vi "VP_RT_base.vi"() -> ()   [LabVIEW 2015] (continued)
                n36 = shared-variable ".\\Interloop communication.lvlib\\System command"(w61) -> ()  [unwired: 1 in, 1 out]
                n37 = local write "System Loop Type"(enum16{"Open Loop", "Closed Loop"}."Closed Loop" ("System Loop Type")) -> ()
              }
            }
            n38 = shared-variable "RT CompactRIO Target\\RT_EPICS_Shared_Variables.lvlib\\2iddVELO:VP:Base_Filename"() -> (w55:string)  [unwired: 1 in, 1 out]
            n39 = local read "EPICS Controller Type"() -> (w54:T2)
            n40 = local write "Fly Scan"(w48) -> ()
            n41 = local write "Controller Type"(w54) -> ()
            n42 = local write "Base name"(w55) -> ()
          }
        }
        "Snake Scan Reference FPGA or EPICS" <- w34
        "EPICS comms error" <- w29
        n43 = shared-variable ".\\Interloop communication.lvlib\\Base Filename"(w26) -> ()  [unwired: 1 in, 1 out]
        n44 = shared-variable ".\\Interloop communication.lvlib\\Command Loop Error"(w29) -> ()  [unwired: 1 in, 1 out]
        n45 = shared-variable ".\\Interloop communication.lvlib\\Fly Scan Flag"(w25) -> ()  [unwired: 1 in, 1 out]
      }
      frame True {
        n46 = shared-variable ".\\Interloop communication.lvlib\\System command"(Command_Enum."Stop System" ("System command")) -> (error out=w70:errorcluster)  [unwired: 1 in]
        n47 = shared-variable ".\\Interloop communication.lvlib\\New Command"(TRUE ("New Command"), error in=w70) -> ()  [unwired: 1 out]
      }
    }
    "Command Loop Iterations" <- w20
  }
  n48 = while {
    shift-right: [w87] -> _
    shift-left: TRUE -> [w88]
    i -> [w76]
    stop <- w80 stop-if-true
    # "Heartbeat Loop"
    n49 = shared-variable ".\\Interloop communication.lvlib\\EPICS command error"() -> (w74:errorcluster)  [unwired: 1 in, 1 out]
    n50 = shared-variable ".\\Interloop communication.lvlib\\Command Loop Error"() -> (w82:errorcluster)  [unwired: 1 in, 1 out]
    n51 = shared-variable ".\\Interloop communication.lvlib\\Readback Loop Error"() -> (w81:errorcluster)  [unwired: 1 in, 1 out]
    n52 = shared-variable ".\\Interloop communication.lvlib\\FPGA startup error"() -> (w79:errorcluster)  [unwired: 1 in, 1 out]
    n53 = shared-variable ".\\Interloop communication.lvlib\\Main Loop Error"() -> (w86:errorcluster)  [unwired: 1 in, 1 out]
    n54 = Not(x=w88) -> (.not. x?=w87:bool)
    "Heartbeat" <- w87
    n55 = call <vilib>:"RT LEDs.vi"("State"=3, "LED Num"=0) -> ("error out"=w75:errorcluster)  [unwired: 4 in, 1 out]
    n56 = Merge Errors(w75, w74, w82, w79, w86, w81) -> (w83:errorcluster)
    n57 = case shown="No Error" w83 {
      selector: w83 -> [w89 w91]
      tunnel: [u32 500 ("millisecond multiple") u32 100 ("millisecond multiple")] -> w85
      tunnel: [w89 w91] -> w84
      frame No Error {
      }
      frame Error {
      }
    }
    "RT error" <- w84
    n58 = local read "Stop System (Careful!!)"() -> (w80:bool)
    n59 = Wait Until Next ms Multiple(millisecond multiple=w85) -> ()  [unwired: 1 out]
    "Heartbeat Loop Iterations" <- w76
  }
  n60 = timed-loop {
    timing: w9 -> [_]
    timing-out: [_] -> w8
    shift-right: [w97] -> _
    shift-left: w4 -> [w94]
    shift-right: [w106] -> _
    shift-left: w2 -> [w98]
    shift-right: [w105] -> _
    shift-left: w1 -> [w99]
    shift-right: [w101] -> _
    shift-left: w3 -> [w102]
    i -> [w103]
    stop <- w108 stop-if-true
    # "Main Loop"
    n61 = node-c288() -> ()  [unwired: 1 in, 1 out]
    n62 = local read "Snake Scan Reference FPGA or EPICS"() -> (w96:enum16{"FPGA Snake Scan", "EPICS Snake Scan"})
    n63 = Format Into String(format string="%s", w94) -> (resulting string=w93:string)  [unwired: 2 in, 1 out]
    n64 = shared-variable "RT CompactRIO Target\\RT_EPICS_Shared_Variables.lvlib\\2iddVELO:VP:RT_State"(w93) -> ()  [unwired: 1 in, 1 out]
    n65 = case shown="\"Update Controller Info\"" w94 {
      tunnel: [w115 w136 w244 w331 w367 w482 w515 w528 w551 w592 w613 w683 w698 w710] -> w107
      tunnel: [FALSE ("Stop") FALSE ("Stop") FALSE ("Stop") FALSE ("Stop") FALSE ("Stop") FALSE ("Stop") FALSE ("Stop") FALSE ("Stop") _ FALSE ("Stop") FALSE ("Stop") FALSE ("Stop") FALSE ("Stop") TRUE ("Stop")] -> w108
      tunnel: [w118 w139 w243 w333 w365 w481 w514 w530 w542 w575 w639 w678 w693 w707] -> w106
      tunnel: [w110 w125 w242 w327 w364 w480 w513 w521 w541 w579 w637 w681 w692 w712] -> w105
      tunnel: w99 -> [w116 w134 w246 w328 w374 w484 w516 w531 w549 w577 w654 w673 w696 w716]
      tunnel: w98 -> [w117 w139 w245 w333 w375 w485 w517 w532 w550 w576 w640 w675 w702 w717]
      tunnel: w102 -> [w115 w136 w244 _ w367 w482 w515 w528 w551 w592 w614 w683 w698 _]
      tunnel: [i64 0 i64 0 i64 0 i64 50 i64 0 i64 0 i64 0 i64 0 i64 0 i64 250 w593 i64 0 i64 0 i64 0] -> w100
      tunnel: w96 -> [_ _ _ _ w361 w477 _ _ _ _ _ _ _ _]
      frame "Initialization", Default {
        n66 = xnode "Invoke Method"("FPGA VI Reference In"=w117, "error in"=w116, "Requested Depth"="Requested Depth") -> ("FPGA VI Reference Out"=w120:refnum<k20>, "error out"=w119:errorcluster, "Actual Depth"=→"Actual Depth":u32)
        n67 = xnode "Read/Write Control"("FPGA VI Reference In"=w120, "error in"=w119, "Datalog Time Period (uSec)"="Datalog Time Period (uSec)", "Datalog Cases"="Datalog Cases") -> ("FPGA VI Reference Out"=w112:refnum<k20>, "error out"=w111:errorcluster)
        n68 = xnode "Read/Write Control"("FPGA VI Reference In"=w112, "error in"=w111) -> ("FPGA VI Reference Out"=w118:refnum<k20>, "error out"=w110:errorcluster, "Wait error"=w109:errorcluster)
        "FPGA wait error" <- w109
        n69 = shared-variable ".\\Interloop communication.lvlib\\FPGA startup error"(w109) -> ()  [unwired: 1 in, 1 out]
      }
      frame "Import Controller coeffs" {
        n70 = case shown="\"PID\"" "Controller Type" {
          tunnel: ["file path soscoeff_zz1 Hinf" "file path soscoeff_zz1 PID"] -> w198
          tunnel: ["file path sos gain SF Controller_zz1 Hinf" "file path sos gain SF Controller_zz1 PID"] -> w196
          tunnel: ["file path soscoeff_yz1 Hinf" "file path soscoeff_zy1 PID"] -> w195
          tunnel: ["file path sos gain SF Controller_yz1 Hinf" "file path sos gain SF Controller_zy1 PID"] -> w194
          tunnel: ["file path soscoeff_yy1 Hinf" "file path soscoeff_yy1 PID"] -> w188
          tunnel: ["file path sos gain SF Controller_yy1 Hinf" "file path sos gain SF Controller_yy1 PID"] -> w187
          tunnel: ["file path soscoeff_zy1 Hinf" "file path soscoeff_yz1 PID"] -> w186
          tunnel: ["file path sos gain SF Controller_zy1 Hinf" "file path sos gain SF Controller_yz1 PID"] -> w185
          tunnel: ["file path soscoeff_xz1 Hinf" "file path soscoeff_zx1 PID"] -> w184
          tunnel: ["file path sos gain SF Controller_xz1 Hinf" "file path sos gain SF Controller_zx1 PID"] -> w183
          tunnel: ["file path soscoeff_xy1 Hinf" "file path soscoeff_yx1 PID"] -> w167
          tunnel: ["file path sos gain SF Controller_xy1 Hinf" "file path sos gain SF Controller_yx1 PID"] -> w166
          tunnel: ["file path sos gain SF Controller_zx1 Hinf" "file path sos gain SF Controller_xz1 PID"] -> w160
          tunnel: ["file path soscoeff_zx1 Hinf" "file path soscoeff_xz1 PID"] -> w159
          tunnel: ["file path sos gain SF Controller_xx1 Hinf" "file path sos gain SF Controller_xx1 PID"] -> w153
          tunnel: ["file path soscoeff_xx1 Hinf" "file path soscoeff_xx1 PID"] -> w152
          tunnel: ["file path soscoeff_yx1 Hinf" "file path soscoeff_xy1 PID"] -> w151
          tunnel: ["file path sos gain SF Controller_yx1 Hinf" "file path sos gain SF Controller_xy1 PID"] -> w150
          frame "H-infinity", Default {
          }
          frame "PID" {
          }
        }
        n71 = call "Read_coeff.vi"("error in (no error)"=w134, "sos gain SF controller file path"=w153, "sos coeff file path"=w152) -> ("b02(2)"=→"b02(2) xx1c":fxp<+/-,64,9>[], "b01(2)"=→"b01(2) xx1c":fxp<+/-,64,9>[], "-a02(2)"=→"-a02(2) xx1c":fxp<+/-,64,9>[], "-a01(2)"=→"-a01(2) xx1c":fxp<+/-,64,9>[], "error out"=w133:errorcluster, "sos gain SF Controller"=→"sos gain SF Controller xx1c":fxp<+/-,42,9>)  [unwired: 3 in]
        n72 = call "Read_coeff.vi"("error in (no error)"=w133, "sos gain SF controller file path"=w166, "sos coeff file path"=w167) -> ("b02(2)"=→"b02(2) xy1c":fxp<+/-,64,9>[], "b01(2)"=→"b01(2) xy1c":fxp<+/-,64,9>[], "-a02(2)"=→"-a02(2) xy1c":fxp<+/-,64,9>[], "-a01(2)"=→"-a01(2) xy1c":fxp<+/-,64,9>[], "error out"=w132:errorcluster, "sos gain SF Controller"=→"sos gain SF Controller xy1c":fxp<+/-,42,9>)  [unwired: 3 in]
        n73 = call "Read_coeff.vi"("error in (no error)"=w132, "sos gain SF controller file path"=w183, "sos coeff file path"=w184) -> ("b02(2)"=→"b02(2) xz1c":fxp<+/-,64,9>[], "b01(2)"=→"b01(2) xz1c":fxp<+/-,64,9>[], "-a02(2)"=→"-a02(2) xz1c":fxp<+/-,64,9>[], "-a01(2)"=→"-a01(2) xz1c":fxp<+/-,64,9>[], "error out"=w131:errorcluster, "sos gain SF Controller"=→"sos gain SF Controller xz1c":fxp<+/-,42,9>)  [unwired: 3 in]
        n74 = call "Read_coeff.vi"("error in (no error)"=w131, "sos gain SF controller file path"=w150, "sos coeff file path"=w151) -> ("b02(2)"=→"b02(2) yx1c":fxp<+/-,64,9>[], "b01(2)"=→"b01(2) yx1c":fxp<+/-,64,9>[], "-a02(2)"=→"-a02(2) yx1c":fxp<+/-,64,9>[], "-a01(2)"=→"-a01(2) yx1c":fxp<+/-,64,9>[], "error out"=w130:errorcluster, "sos gain SF Controller"=→"sos gain SF Controller yx1c":fxp<+/-,42,9>)  [unwired: 3 in]
        n75 = call "Read_coeff.vi"("error in (no error)"=w130, "sos gain SF controller file path"=w187, "sos coeff file path"=w188) -> ("b02(2)"=→"b02(2) yy1c":fxp<+/-,64,9>[], "b01(2)"=→"b01(2) yy1c":fxp<+/-,64,9>[], "-a02(2)"=→"-a02(2) yy1c":fxp<+/-,64,9>[], "-a01(2)"=→"-a01(2) yy1c":fxp<+/-,64,9>[], "error out"=w129:errorcluster, "sos gain SF Controller"=→"sos gain SF Controller yy1c":fxp<+/-,42,9>)  [unwired: 3 in]
        n76 = call "Read_coeff.vi"("error in (no error)"=w129, "sos gain SF controller file path"=w194, "sos coeff file path"=w195) -> ("b02(2)"=→"b02(2) yz1c":fxp<+/-,64,9>[], "b01(2)"=→"b01(2) yz1c":fxp<+/-,64,9>[], "-a02(2)"=→"-a02(2) yz1c":fxp<+/-,64,9>[], "-a01(2)"=→"-a01(2) yz1c":fxp<+/-,64,9>[], "error out"=w128:errorcluster, "sos gain SF Controller"=→"sos gain SF Controller yz1c":fxp<+/-,42,9>)  [unwired: 3 in]
        n77 = call "Read_coeff.vi"("error in (no error)"=w128, "sos gain SF controller file path"=w160, "sos coeff file path"=w159) -> ("b02(2)"=→"b02(2) zx1c":fxp<+/-,64,9>[], "b01(2)"=→"b01(2) zx1c":fxp<+/-,64,9>[], "-a02(2)"=→"-a02(2) zx1c":fxp<+/-,64,9>[], "-a01(2)"=→"-a01(2) zx1c":fxp<+/-,64,9>[], "error out"=w127:errorcluster, "sos gain SF Controller"=→"sos gain SF Controller zx1c":fxp<+/-,42,9>)  [unwired: 3 in]
        n78 = call "Read_coeff.vi"("error in (no error)"=w127, "sos gain SF controller file path"=w185, "sos coeff file path"=w186) -> ("b02(2)"=→"b02(2) zy1c":fxp<+/-,64,9>[], "b01(2)"=→"b01(2) zy1c":fxp<+/-,64,9>[], "-a02(2)"=→"-a02(2) zy1c":fxp<+/-,64,9>[], "-a01(2)"=→"-a01(2) zy1c":fxp<+/-,64,9>[], "error out"=w126:errorcluster, "sos gain SF Controller"=→"sos gain SF Controller zy1c":fxp<+/-,42,9>)  [unwired: 3 in]
        n79 = call "Read_coeff.vi"("error in (no error)"=w126, "sos gain SF controller file path"=w196, "sos coeff file path"=w198) -> ("b02(2)"=→"b02(2) zz1c":fxp<+/-,64,9>[], "b01(2)"=→"b01(2) zz1c":fxp<+/-,64,9>[], "-a02(2)"=→"-a02(2) zz1c":fxp<+/-,64,9>[], "-a01(2)"=→"-a01(2) zz1c":fxp<+/-,64,9>[], "error out"=w125:errorcluster, "sos gain SF Controller"=→"sos gain SF Controller zz1c":fxp<+/-,42,9>)  [unwired: 3 in]
        "Coeff file import error" <- w125
      }
      frame "Update Controller Info" {
        n80 = local read "sos gain SF Controller yy1c"() -> (w305:fxp<+/-,42,9>)
        n81 = local read "sos gain SF Controller yz1c"() -> (w254:fxp<+/-,42,9>)
        n82 = local read "sos gain SF Controller yx1c"() -> (w293:fxp<+/-,42,9>)
        n83 = local read "sos gain SF Controller xy1c"() -> (w279:fxp<+/-,42,9>)
        n84 = local read "sos gain SF Controller zy1c"() -> (w284:fxp<+/-,42,9>)
        n85 = local read "sos gain SF Controller xz1c"() -> (w268:fxp<+/-,42,9>)
        n86 = local read "sos gain SF Controller xx1c"() -> (w310:fxp<+/-,42,9>)
        n87 = local read "sos gain SF Controller zz1c"() -> (w303:fxp<+/-,42,9>)
        n88 = local read "sos gain SF Controller zx1c"() -> (w289:fxp<+/-,42,9>)
        n89 = local read "-a01(2) yy1c"() -> (w309:fxp<+/-,64,9>[])
        n90 = local read "-a02(2) yy1c"() -> (w308:fxp<+/-,64,9>[])
        n91 = local read "-a01(2) yz1c"() -> (w273:fxp<+/-,64,9>[])
        n92 = local read "-a02(2) yz1c"() -> (w274:fxp<+/-,64,9>[])
        n93 = local read "-a01(2) yx1c"() -> (w294:fxp<+/-,64,9>[])
        n94 = local read "-a02(2) yx1c"() -> (w290:fxp<+/-,64,9>[])
        n95 = local read "-a01(2) xy1c"() -> (w275:fxp<+/-,64,9>[])
        n96 = local read "-a02(2) xy1c"() -> (w276:fxp<+/-,64,9>[])
        n97 = local read "-a01(2) zy1c"() -> (w280:fxp<+/-,64,9>[])
        n98 = local read "-a02(2) zy1c"() -> (w281:fxp<+/-,64,9>[])
        n99 = local read "-a01(2) xz1c"() -> (w272:fxp<+/-,64,9>[])
        n100 = local read "-a02(2) xz1c"() -> (w271:fxp<+/-,64,9>[])
        n101 = local read "-a01(2) xx1c"() -> (w314:fxp<+/-,64,9>[])
        n102 = local read "-a02(2) xx1c"() -> (w313:fxp<+/-,64,9>[])
        n103 = local read "-a01(2) zz1c"() -> (w304:fxp<+/-,64,9>[])
        n104 = local read "-a02(2) zz1c"() -> (w300:fxp<+/-,64,9>[])
        n105 = local read "-a01(2) zx1c"() -> (w285:fxp<+/-,64,9>[])
        n106 = local read "-a02(2) zx1c"() -> (w286:fxp<+/-,64,9>[])
        n107 = local read "b01(2) yy1c"() -> (w307:fxp<+/-,64,9>[])
        n108 = local read "b02(2) yy1c"() -> (w306:fxp<+/-,64,9>[])
        n109 = local read "b01(2) yz1c"() -> (w248:fxp<+/-,64,9>[])
        n110 = local read "b02(2) yz1c"() -> (w247:fxp<+/-,64,9>[])
        n111 = local read "b01(2) yx1c"() -> (w291:fxp<+/-,64,9>[])
        n112 = local read "b02(2) yx1c"() -> (w292:fxp<+/-,64,9>[])
        n113 = local read "b01(2) xy1c"() -> (w277:fxp<+/-,64,9>[])
        n114 = local read "b02(2) xy1c"() -> (w278:fxp<+/-,64,9>[])
        n115 = local read "b01(2) zy1c"() -> (w282:fxp<+/-,64,9>[])
        n116 = local read "b02(2) zy1c"() -> (w283:fxp<+/-,64,9>[])
        n117 = local read "b01(2) xz1c"() -> (w270:fxp<+/-,64,9>[])
        n118 = local read "b02(2) xz1c"() -> (w269:fxp<+/-,64,9>[])
        n119 = local read "b01(2) xx1c"() -> (w312:fxp<+/-,64,9>[])
        n120 = local read "b02(2) xx1c"() -> (w311:fxp<+/-,64,9>[])
        n121 = local read "b01(2) zz1c"() -> (w301:fxp<+/-,64,9>[])
        n122 = local read "b02(2) zz1c"() -> (w302:fxp<+/-,64,9>[])
        n123 = local read "b01(2) zx1c"() -> (w287:fxp<+/-,64,9>[])
        n124 = local read "b02(2) zx1c"() -> (w288:fxp<+/-,64,9>[])
        n125 = Or(x="Optics Z Reset", y="Reset All") -> (x .or. y?=w267:bool)
        n126 = Or(x="Sample Z Reset", y="Reset All") -> (x .or. y?=w264:bool)
        n127 = Or(x="Optics X Reset", y="Reset All") -> (x .or. y?=w298:bool)
        n128 = Or(x="Optics Y Reset", y="Reset All") -> (x .or. y?=w296:bool)
        n129 = Or(x="Sample X Reset", y="Reset All") -> (x .or. y?=w266:bool)
        n130 = Or(x="Sample Y Reset", y="Reset All") -> (x .or. y?=w265:bool)
        n131 = xnode "Read/Write Control"("FPGA VI Reference In"=w245, "error in"=w246, "Wait timer (ms)"="FPGA Wait Timer (ms)", "Controller Time Period (uSec)"="Controller Time Period (uSec)", "Controller Output Time Period (uSec)"="Controller Output Time Period (uSec)", "System Loop Type"="System Loop Type", "Controller Output Upper Limit"="Controller Output Upper Limit", "Controller Output Lower Limit"="Controller Output Lower Limit", "X-Stage nm to V Scaling"="X-Stage nm to V Scaling", "X-Stage Scaling Direction"="X-Stage Scaling Direction", "Y-Stage nm to V Scaling"="Y-Stage nm to V Scaling", "Z-Stage nm to V Scaling"="Z-Stage nm to V Scaling", "Plant Output Time Period (uSec)"="Plant Output Time Period (uSec)", "Reset Optics X"=w298, "Reset Optics Y"=w296, "Reset Optics Z"=w267, "Reset Sample X"=w266, "Reset Sample Y"=w265, "Reset Sample Z"=w264, "Optics X Stage Resolution (nm)"="Optics X Stage Resolution (nm)", "Optics Y Stage Resolution (nm)"="Optics Y Stage Resolution (nm)", "Optics Z Stage Resolution (nm)"="Optics Z Stage Resolution (nm)", "Sample X Stage Resolution (nm)"="Sample X Stage Resolution (nm)", "Sample Y Stage Resolution (nm)"="Sample Y Stage Resolution (nm)", "Sample Z Stage Resolution (nm)"="Sample Z Stage Resolution (nm)", "Scaling mV to V"="Scaling mV to V", "-a01(2) xx1"=w314, "-a02(2) xx1"=w313, "b01(2) xx1"=w312, "b02(2) xx1"=w311, "sos gain SF Controller xx1"=w310, "-a01(2) yy1"=w309, "-a02(2) yy1"=w308, "b01(2) yy1"=w307, "b02(2) yy1"=w306, "sos gain SF Controller yy1"=w305, "-a01(2) zz1"=w304, "-a02(2) zz1"=w300, "b01(2) zz1"=w301, "b02(2) zz1"=w302, "sos gain SF Controller zz1"=w303, "-a01(2) yx1"=w294, "-a02(2) yx1"=w290, "b01(2) yx1"=w291, "b02(2) yx1"=w292, "sos gain SF Controller yx1"=w293, "-a01(2) zx1"=w285, "-a02(2) zx1"=w286, "b01(2) zx1"=w287, "b02(2) zx1"=w288, "sos gain SF Controller zx1"=w289, "-a01(2) xy1"=w275, "-a02(2) xy1"=w276, "b01(2) xy1"=w277, "b02(2) xy1"=w278, "sos gain SF Controller xy1"=w279, "-a01(2) zy1"=w280, "-a02(2) zy1"=w281, "b01(2) zy1"=w282, "b02(2) zy1"=w283, "sos gain SF Controller zy1"=w284, "-a01(2) xz1"=w272, "-a02(2) xz1"=w271, "b01(2) xz1"=w270, "b02(2) xz1"=w269, "sos gain SF Controller xz1"=w268, "-a01(2) yz1"=w273, "-a02(2) yz1"=w274, "b01(2) yz1"=w248, "b02(2) yz1"=w247, "sos gain SF Controller yz1"=w254, "Analog Input Time Period (uSec)"="Analog Input Time Period (uSec)", "Optics and or Sample Stage"="Optics and or Sample Stage", "Y-Stage Scaling Direction"="Y-Stage Scaling Direction", "Z-Stage Scaling Direction"="Z-Stage Scaling Direction") -> ("FPGA VI Reference Out"=w243:refnum<k20>, "error out"=w242:errorcluster)
      }
      frame "Wait" {
        n132 = shared-variable ".\\Interloop communication.lvlib\\New Command"() -> (w332:bool, error out=w330:errorcluster)  [unwired: 1 in]
        n133 = case shown="True" w332 {
          tunnel: [w335 w336] -> w331
          tunnel: w330 -> [_ w340]
          tunnel: w328 -> [w334 w338]
          tunnel: [w334 w337] -> w327
          frame False {
            w335 = T11[] [enum."Wait"] items=["Initialization", "Import Controller coeffs", "Update Controller Info", "Wait", "Update Reference Info", "Update Detector Trigger Info", "Update Datalog Info", "Check FPGA Status", "Pre-Scan", "Start Scan", "Step Scanning", "Fly Scanning", "End Scan", "Restart FPGA", "Stop FPGA"]
          }
          frame True {
            n134 = shared-variable ".\\Interloop communication.lvlib\\System command"() -> (w339:T8)  [unwired: 1 in, 1 out]
            "Last Command Executed" <- w339
            n135 = case shown="\"Scan\"" w339 {
              tunnel: [w344 w347 w350 w353 w356 w360] -> w336
              tunnel: w338 -> [w343 w346 w349 w352 w355 w359]
              tunnel: [w342 w345 w348 w351 w354 w358] -> w337
              frame "Re-Initialize ", Default {
                w344 = T11[] [enum."Initialization", enum."Import Controller coeffs", enum."Update Controller Info", enum."Wait"] items=["Initialization", "Import Controller coeffs", "Update Controller Info", "Wait", "Update Reference Info", "Update Detector Trigger Info", "Update Datalog Info", "Check FPGA Status", "Pre-Scan", "Start Scan", "Step Scanning", "Fly Scanning", "End Scan", "Restart FPGA", "Stop FPGA"]
                n136 = call <vilib>:"Clear Errors.vi"("error in (no error)"=w343) -> ("error out"=w342:errorcluster)  [unwired: 5 in, 1 out]
              }
              frame "Update Scan Settings" {
                w347 = T11[] [enum."Update Reference Info", enum."Update Detector Trigger Info", enum."Update Datalog Info", enum."Wait"] items=["Initialization", "Import Controller coeffs", "Update Controller Info", "Wait", "Update Reference Info", "Update Detector Trigger Info", "Update Datalog Info", "Check FPGA Status", "Pre-Scan", "Start Scan", "Step Scanning", "Fly Scanning", "End Scan", "Restart FPGA", "Stop FPGA"]
                n137 = call <vilib>:"Clear Errors.vi"("error in (no error)"=w346) -> ("error out"=w345:errorcluster)  [unwired: 5 in, 1 out]
              }
              frame "Scan" {
                w350 = T11[] [enum."Update Reference Info", enum."Update Detector Trigger Info", enum."Update Datalog Info", enum."Pre-Scan", enum."Start Scan", enum."Fly Scanning", enum."End Scan", enum."Wait"] items=["Initialization", "Import Controller coeffs", "Update Controller Info", "Wait", "Update Reference Info", "Update Detector Trigger Info", "Update Datalog Info", "Check FPGA Status", "Pre-Scan", "Start Scan", "Step Scanning", "Fly Scanning", "End Scan", "Restart FPGA", "Stop FPGA"]
                n138 = call <vilib>:"Clear Errors.vi"("error in (no error)"=w349) -> ("error out"=w348:errorcluster)  [unwired: 5 in, 1 out]
              }
              frame "Stop Scan" {
                w353 = T11[] [enum."End Scan", enum."Wait"] items=["Initialization", "Import Controller coeffs", "Update Controller Info", "Wait", "Update Reference Info", "Update Detector Trigger Info", "Update Datalog Info", "Check FPGA Status", "Pre-Scan", "Start Scan", "Step Scanning", "Fly Scanning", "End Scan", "Restart FPGA", "Stop FPGA"]
                n139 = call <vilib>:"Clear Errors.vi"("error in (no error)"=w352) -> ("error out"=w351:errorcluster)  [unwired: 5 in, 1 out]
              }
              frame "Restart FPGA" {
                w356 = T11[] [enum."Restart FPGA", enum."Initialization", enum."Import Controller coeffs", enum."Update Controller Info", enum."Wait"] items=["Initialization", "Import Controller coeffs", "Update Controller Info", "Wait", "Update Reference Info", "Update Detector Trigger Info", "Update Datalog Info", "Check FPGA Status", "Pre-Scan", "Start Scan", "Step Scanning", "Fly Scanning", "End Scan", "Restart FPGA", "Stop FPGA"]
                n140 = call <vilib>:"Clear Errors.vi"("error in (no error)"=w355) -> ("error out"=w354:errorcluster)  [unwired: 5 in, 1 out]
              }
              frame "Stop System" {
                w360 = T11[] [enum."Stop FPGA"] items=["Initialization", "Import Controller coeffs", "Update Controller Info", "Wait", "Update Reference Info", "Update Detector Trigger Info", "Update Datalog Info", "Check FPGA Status", "Pre-Scan", "Start Scan", "Step Scanning", "Fly Scanning", "End Scan", "Restart FPGA", "Stop FPGA"]
                n141 = call <vilib>:"Clear Errors.vi"("error in (no error)"=w359) -> ("error out"=w358:errorcluster)  [unwired: 5 in, 1 out]
                n142 = local write "Stop System (Careful!!)"(TRUE ("Stop")) -> ()
              }
            }
            n143 = shared-variable ".\\Interloop communication.lvlib\\New Command"(FALSE ("New Command"), error in=w340) -> ()  [unwired: 1 out]
          }
        }
      }
      frame "Update Reference Info" {
        w427 = errorcluster {"status"=FALSE, "code"=0, "source"=""}  # error in (no error)
        w430 = errorcluster {"status"=FALSE, "code"=0, "source"=""}  # error in (no error)
        w444 = errorcluster {"status"=FALSE, "code"=0, "source"=""}  # error in (no error)
        w423 = 40000000.0  # FPGA clock rate (Hz)
        n144 = local read "Measured Z Reference Time Period (Ticks)"() -> (w366:u32)
        n145 = case shown="\"EPICS Snake Scan\"" w361 {
          tunnel: ["X Ramp Start (nm)" w460] -> w382
          tunnel: ["X Ramp End (nm)" w459] -> w381
          tunnel: ["Y Ramp Start (nm)" w458] -> w380
          tunnel: ["Y Ramp End (nm)" w457] -> w379
          tunnel: ["Y Step Size (nm)" w461] -> w378
          tunnel: ["X Step Size (nm)" w464] -> w377
          tunnel: [w452 w462] -> w376
          tunnel: ["Y Step Size (nm)" w461] -> w373
          tunnel: ["X Ramp Start (nm)" w460] -> w372
          tunnel: ["X Ramp End (nm)" w459] -> w371
          tunnel: ["Y Ramp Start (nm)" w458] -> w370
          tunnel: ["Y Ramp End (nm)" w457] -> w369
          frame "FPGA Snake Scan", Default {
            n146 = local read "DT Frequency (Hz)"() -> (w452:dbl)
          }
          frame "EPICS Snake Scan" {
            w463 = fxp<+/-,16,16> 0.0 ("fixed-point type")
            n147 = shared-variable "RT CompactRIO Target\\RT_EPICS_Shared_Variables.lvlib\\2iddVELO:VP:Trigger_Freq_Hz"() -> (w462:dbl)  [unwired: 1 in, 1 out]
            "2iddVELO:VP:Trigger_Freq_Hz" <- w462
            n148 = shared-variable "RT CompactRIO Target\\RT_EPICS_Shared_Variables.lvlib\\2iddVELO:VP:Y_Step_Size_nm"() -> (w466:dbl)  [unwired: 1 in, 1 out]
            "2iddVELO:VP:Y_Step_Size_nm" <- w466
            n149 = shared-variable "RT CompactRIO Target\\RT_EPICS_Shared_Variables.lvlib\\2iddVELO:VP:X_Step_Size_nm"() -> (w465:dbl)  [unwired: 1 in, 1 out]
            "2iddVELO:VP:X_Step_Size_nm" <- w465
            n150 = shared-variable "RT CompactRIO Target\\RT_EPICS_Shared_Variables.lvlib\\2iddVELO:VP:Y_Start_nm"() -> (w467:dbl)  [unwired: 1 in, 1 out]
            n151 = shared-variable "RT CompactRIO Target\\RT_EPICS_Shared_Variables.lvlib\\2iddVELO:VP:Y_End_nm"() -> (w456:dbl)  [unwired: 1 in, 1 out]
            n152 = shared-variable "RT CompactRIO Target\\RT_EPICS_Shared_Variables.lvlib\\2iddVELO:VP:X_Start_nm"() -> (w469:dbl)  [unwired: 1 in, 1 out]
            "2iddVELO:VP:X_Start_nm" <- w469
            n153 = shared-variable "RT CompactRIO Target\\RT_EPICS_Shared_Variables.lvlib\\2iddVELO:VP:X_End_nm"() -> (w468:dbl)  [unwired: 1 in, 1 out]
            "2iddVELO:VP:X_End_nm" <- w468
            n154 = Negate(x=w456) -> (-x=w455:dbl)
            "2iddVELO:VP:Y_End_nm" <- w455
            n155 = Negate(x=w467) -> (-x=w454:dbl)
            "2iddVELO:VP:Y_Start_nm" <- w454
            n156 = To Fixed-Point(fixed-point type=w463, number=w469) -> (fixed-point=w460:fxp<+/-,16,16>)
            n157 = To Fixed-Point(fixed-point type=w463, number=w468) -> (fixed-point=w459:fxp<+/-,16,16>)
            n158 = To Fixed-Point(fixed-point type=w463, number=w454) -> (fixed-point=w458:fxp<+/-,16,16>)
            n159 = To Fixed-Point(fixed-point type=w463, number=w455) -> (fixed-point=w457:fxp<+/-,16,16>)
            n160 = To Fixed-Point(fixed-point type=w463, number=w466) -> (fixed-point=w461:fxp<+/-,16,16>)
            n161 = To Fixed-Point(fixed-point type=w463, number=w465) -> (fixed-point=w464:fxp<+/-,16,16>)
          }
        }
        n162 = local read "Y Ramp Period (usec)"() -> (w384:fxp<+,24,24>)
        n163 = shared-variable ".\\Interloop communication.lvlib\\Fly Scan Flag"() -> (w368:bool)  [unwired: 1 in, 1 out]
        n164 = case shown="\"Sawtooth Wave\"" "Z Reference Wave Selection" {
          tunnel: "Z frequency (Hz)" -> [w470 w471 w473 w475 w476]
          tunnel: [w470 w471 w472 w475 w476] -> w405
          tunnel: w366 -> [_ _ w474 _ _]
          frame "Constant", Default {
          }
          frame "Sine Wave" {
          }
          frame "Sawtooth Wave" {
            n165 = Multiply(x=w474, y=w473) -> (x*y=w472:dbl)
          }
          frame "Square Wave" {
          }
          frame "Filtered White Noise" {
          }
        }
        n166 = call <vilib>:"Normalize Signal Generation Parameters.vi"("frequency (Hz)"="X frequency (Hz)", "FPGA clock rate (Hz)"=w423, "phase offset (deg)"="X phase offset (deg)", "error in (no error)"=w444) -> ("frequency (periods/tick)"=w443:fxp<+,32,0>, "phase offset (periods)"=w433:fxp<+,32,0>, "error out"=→"error out (Sig Gen)":errorcluster)  [unwired: 6 in, 3 out]
        "X frequency (periods/tick)" <- w443
        "X phase offset (periods)" <- w433
        n167 = call <vilib>:"Normalize Signal Generation Parameters.vi"("frequency (Hz)"="Y frequency (Hz)", "FPGA clock rate (Hz)"=w423, "phase offset (deg)"="Y phase offset (deg)", "error in (no error)"=w430) -> ("frequency (periods/tick)"=w426:fxp<+,32,0>, "phase offset (periods)"=w425:fxp<+,32,0>, "error out"=→"error out (Sig Gen) 2":errorcluster)  [unwired: 6 in, 3 out]
        "Y frequency (periods/tick)" <- w426
        "Y phase offset (periods)" <- w425
        n168 = call <vilib>:"Normalize Signal Generation Parameters.vi"("frequency (Hz)"=w405, "FPGA clock rate (Hz)"=w423, "phase offset (deg)"="Z phase offset (deg)", "error in (no error)"=w427) -> ("frequency (periods/tick)"=w424:fxp<+,32,0>, "phase offset (periods)"=w416:fxp<+,32,0>, "error out"=→"error out (Sig Gen) 3":errorcluster)  [unwired: 6 in, 3 out]
        "Z frequency (periods/tick)" <- w424
        "Z phase offset (periods)" <- w416
        n169 = local read "X Ramp Period (usec)"() -> (w383:fxp<+,24,24>)
        n170 = xnode "Read/Write Control"("FPGA VI Reference In"=w375, "error in"=w374, "X Reference Time Period (uSec)"="X Reference Time Period (uSec)", "Y Reference Time Period (uSec)"="Y Reference Time Period (uSec)", "Z Reference Time Period (uSec)"="Z Reference Time Period (uSec)", "X Reference Wave Selection"="X Reference Wave Selection", "Y Reference Wave Selection"="Y Reference Wave Selection", "Z Reference Wave Selection"="Z Reference Wave Selection", "X Reference Reset"="X Reference Reset", "Y Reference Reset"="Y Reference Reset", "Z Reference Reset"="Z Reference Reset", "X Reference Amplitude (nm)"="X Reference Amplitude (nm)", "Y Reference Amplitude (nm)"="Y Reference Amplitude (nm)", "Z Reference Amplitude (nm)"="Z Reference Amplitude (nm)", "X Frequency (periods/tick)"=w443, "X Phase Offset (periods)"=w433, "Y Frequency (periods/tick)"=w426, "Y Phase Offset (periods)"=w425, "Z Frequency (periods/tick)"=w424, "Z Phase Offset (periods)"=w416, "X Reference DC Offset (nm)"="X Reference DC Offset (nm)", "Y Reference DC Offset (nm)"="Y Reference DC Offset (nm)", "Z Reference DC Offset (nm)"="Z Reference DC Offset (nm)", "X White Noise Amplitude"="X White Noise Amplitude", "X White Noise Seed"="X White Noise Seed", "Y White Noise Amplitude"="Y White Noise Amplitude", "Y White Noise Seed"="Y White Noise Seed", "Z White Noise Amplitude"="Z White Noise Amplitude", "Z White Noise Seed"="Z White Noise Seed", "Mod 3 AI0 V to nm Scaling"="Mod 3 AI0 V to nm Scaling", "Mod 3 AI1 V to nm Scaling"="Mod 3 AI1 V to nm Scaling", "Mod 3 AI2 V to nm Scaling"="Mod 3 AI2 V to nm Scaling", "X Ramp Period (usec)"=w383, "X Ramp Start (nm)"=w382, "X Ramp End (nm)"=w381, "X Start Marker (nm)"="X Start Marker (nm)", "Fly Scan"=w368, "Y Ramp Period (usec)"=w384, "Y Ramp Start (nm)"=w380, "Y Ramp End (nm)"=w379, "Y Ramp Drop Size (nm)"=w378, "Y Start Marker (nm)"="Y Start Marker (nm)") -> ("FPGA VI Reference Out"=w365:refnum<k20>, "error out"=w364:errorcluster)
        n171 = Subtract(x=w370, y=w369) -> (x-y=w400:fxp<+/-,17,17>)
        n172 = Subtract(x=w372, y=w371) -> (x-y=w398:fxp<+/-,17,17>)
        n173 = Absolute Value(x=w400) -> (abs(x)=w391:fxp<+,16,16>)
        n174 = Absolute Value(x=w398) -> (abs(x)=w397:fxp<+,16,16>)
        n175 = Divide(x=w397, y=w377) -> (x/y=w395:fxp<+/-,33,17>)
        "# of Points per Line" <- w395
        n176 = Divide(x=w395, y=w376) -> (x/y=w387:dbl)
        "sec per line" <- w387
        n177 = Divide(x=w391, y=w373) -> (x/y=w392:fxp<+/-,33,17>)
        n178 = Add(x=w392, y=fxp<+,16,16> 1.0) -> (x+y=w386:fxp<+/-,34,18>)
        "# of Hor Lines" <- w386
        n179 = Multiply(x=w387, y=1000000.0) -> (x*y=w390:dbl)
        "X Ramp Period DBL (usec)" <- w390
        n180 = Reciprocal(x=w387) -> (1/x=→"line per sec (Hz)":dbl)
        n181 = To Fixed-Point(fixed-point type=fxp<+,24,24> 0.0, number=w390) -> (fixed-point=→"X Ramp Period (usec)" →"Y Ramp Period (usec)":fxp<+,24,24>)
        n182 = Multiply(x=w387, y=w386) -> (x*y=→"Total Scan Time (sec)":dbl)
        n183 = Multiply(x=w386, y=w395) -> (x*y=→"# Total Trigger Points":fxp<+/-,64,34>)
      }
      frame "Update Detector Trigger Info" {
        w491 = 40000000.0  # FPGA clock rate (Hz)
        w493 = errorcluster {"status"=FALSE, "code"=0, "source"=""}  # error in (no error)
        n184 = case shown="\"EPICS Snake Scan\"" w477 {
          tunnel: ["DT Frequency (Hz)" w510] -> w492
          tunnel: ["DT duty cycle (%)" w509] -> w486
          frame "FPGA Snake Scan", Default {
          }
          frame "EPICS Snake Scan" {
            n185 = shared-variable "RT CompactRIO Target\\RT_EPICS_Shared_Variables.lvlib\\2iddVELO:VP:Trig_DutyCycle_Per"() -> (w509:dbl)  [unwired: 1 in, 1 out]
            "2iddVELO:VP:Trig_DutyCycle_Per" <- w509
            n186 = shared-variable "RT CompactRIO Target\\RT_EPICS_Shared_Variables.lvlib\\2iddVELO:VP:Trigger_Freq_Hz"() -> (w510:dbl)  [unwired: 1 in, 1 out]
          }
        }
        "Trigger Frequency (Hz)" <- w492
        "Trigger Duty Cycle (%)" <- w486
        n187 = call <vilib>:"Normalize Signal Generation Parameters.vi"("frequency (Hz)"=w492, "FPGA clock rate (Hz)"=w491, "phase offset (deg)"="DT phase offset (deg)", "duty cycle (%)"=w486, "error in (no error)"=w493) -> ("frequency (periods/tick)"=w489:fxp<+,32,0>, "phase offset (periods)"=w488:fxp<+,32,0>, "duty cycle (periods)"=w487:fxp<+,32,0>, "error out"=→"error out (Sig Gen) 4":errorcluster)  [unwired: 5 in, 2 out]
        "DT Frequency (periods/tick)" <- w489
        "DT Phase Offset (periods)" <- w488
        "DT Duty Cycle (periods)" <- w487
        n188 = xnode "Read/Write Control"("FPGA VI Reference In"=w485, "error in"=w484, "Detector Trigger Time Period (uSec)"="Detector Trigger Time Period (uSec)", "Trigger Generation Time Period (uSec)"="Trigger Generation Time Period (uSec)", "Detector Trigger Lower Limit (V)"="Detector Trigger Lower Limit (V)", "Detector Trigger Upper Limit (V)"="Detector Trigger Upper Limit (V)", "Trigger High Period (usec)"="Trigger High Period (usec)", "Trigger Low Period (usec)"="Trigger Low Period (usec)", "Trigger High Level (V)"="Trigger High Level (V)", "Trigger Low Level (V)"="Trigger Low Level (V)", "Trigger Wave Generator"="Trigger Wave Generator", "DT Reference Amplitude (V)"="DT Reference Amplitude (V)", "DT Reference DC Offset (V)"="DT Reference DC Offset (V)", "DT Frequency (periods/tick)"=w489, "DT Phase Offset (periods)"=w488, "DT Reset"="DT Reset", "DT Duty Cycle (periods)"=w487, "Data Trigger Time Period (uSec)"="Data Trigger Time Period (uSec)") -> ("FPGA VI Reference Out"=w481:refnum<k20>, "error out"=w480:errorcluster)
      }
      frame "Update Datalog Info" {
        n189 = local read "Datalog Time Period (uSec)"() -> (w520:u32)
        n190 = local read "Datalog Cases"() -> (w519:T3)
        n191 = xnode "Read/Write Control"("FPGA VI Reference In"=w517, "error in"=w516, "Datalog Time Period (uSec)"=w520, "Datalog Cases"=w519, "Timeout FPGA FIFO1"="Timeout FPGA FIFO1") -> ("FPGA VI Reference Out"=w514:refnum<k20>, "error out"=w513:errorcluster)
      }
      frame "Check FPGA Status" {
        n192 = xnode "Read/Write Control"("FPGA VI Reference In"=w532, "error in"=w531) -> ("FPGA VI Reference Out"=w530:refnum<k20>, "error out"=w529:errorcluster, "FPGA error monitor"=w535:errorcluster, "End Run Error"=w534:errorcluster, "FIFO Timed Out?"=→"FIFO Timed Out?":bool, "stop case"=w524:bool, "FIFO Timed Out"=w525:bool)
        "FPGA error monitor" <- w535
        "FPGA end run error" <- w534
        "stop case" <- w524
        "FIFO Timed Out" <- w525
        n193 = case shown="True" w524 {
          tunnel: [errorcluster {"status"=FALSE, "code"=0, "source"=""} ("error constant") errorcluster {"status"=TRUE, "code"=7002, "source"="FPGA stop case encountered"} ("error constant")] -> w522
          frame False {
          }
          frame True {
          }
        }
        n194 = case shown="True" w525 {
          tunnel: [errorcluster {"status"=FALSE, "code"=0, "source"=""} ("error constant") errorcluster {"status"=TRUE, "code"=7001, "source"="FPGA FIFO timed out"} ("error constant")] -> w523
          frame False {
          }
          frame True {
          }
        }
        n195 = Merge Errors(w529, w535, w534, w522, w523) -> (w521:errorcluster)
      }
      frame "Pre-Scan" {
        n196 = flat-sequence {
          tunnel: w550 -> [w557]
          tunnel: w549 -> [w556]
          tunnel: [w553] -> w548
          tunnel: [w552] -> w546
          tunnel: w548 -> [w563]
          tunnel: [w563] -> w547
          tunnel: w546 -> [w562]
          tunnel: [w562] -> w545
          tunnel: w547 -> [w567]
          tunnel: w545 -> [w566]
          tunnel: [w565] -> w544
          tunnel: [w564] -> w543
          tunnel: w544 -> [w574]
          tunnel: w543 -> [w573]
          tunnel: [w570] -> w542
          tunnel: [w569] -> w541
          frame #0 {
            w554 = TRUE
            n197 = xnode "Read/Write Control"("FPGA VI Reference In"=w557, "error in"=w556, "Reset Optics X"=w554, "Reset Optics Y"=w554, "Reset Optics Z"=w554, "Reset Sample X"=w554, "Reset Sample Y"=w554, "Reset Sample Z"=w554, "System Loop Type"=enum16{"Open Loop", "Closed Loop"}."Open Loop", "New FPGA command"=TRUE, "FPGA command"=enum16{"Start Scan", "Shutdown"}."Start Scan", "Fly Scan"=FALSE) -> ("FPGA VI Reference Out"=w553:refnum<k20>, "error out"=w552:errorcluster)
          }
          frame #1 {
            n198 = Wait (ms)(milliseconds to wait="Pre-Scan pause (ms)") -> ()  [unwired: 1 out]
          }
          frame #2 {
            n199 = xnode "Read/Write Control"("FPGA VI Reference In"=w567, "error in"=w566, "stop case"=TRUE) -> ("FPGA VI Reference Out"=w565:refnum<k20>, "error out"=w564:errorcluster)
          }
          frame #3 {
            w571 = FALSE ("Reset Optics X")
            n200 = local read "System Loop Type"() -> (w572:enum16{"Open Loop", "Closed Loop"})
            n201 = xnode "Read/Write Control"("FPGA VI Reference In"=w574, "error in"=w573, "Reset Optics X"=w571, "Reset Optics Y"=w571, "Reset Optics Z"=w571, "Reset Sample X"=w571, "Reset Sample Y"=w571, "Reset Sample Z"=w571, "System Loop Type"=w572) -> ("FPGA VI Reference Out"=w570:refnum<k20>, "error out"=w569:errorcluster)
          }
        }
      }
      frame "Start Scan" {
        n202 = shared-variable ".\\Interloop communication.lvlib\\Base Filename"() -> (w580:string)  [unwired: 1 in, 1 out]
        n203 = String To Path(string="cRIO data dir") -> (path=w581:path)
        "cRIO path" <- w581
        n204 = call "Data_Write.vi"("Destination dir"=w581, "error initialize"=w577, "Base name"=w580, "Command List"=Data_Write_Control."Initialize") -> ("error out"=w578:errorcluster, "Path"=w589:path)  [unwired: 4 in]
        n205 = Strip Path(path=w589) -> (stripped path=→"Output path":path, name=→"Output filename":string)
        n206 = shared-variable ".\\Interloop communication.lvlib\\Fly Scan Flag"() -> (w584:bool)  [unwired: 1 in, 1 out]
        n207 = xnode "Read/Write Control"("FPGA VI Reference In"=w576, "error in"=w578, "New FPGA command"=TRUE, "FPGA command"=enum16{"Start Scan", "Shutdown"}."Start Scan", "Fly Scan"=w584) -> ("FPGA VI Reference Out"=w575:refnum<k20>, "error out"=w579:errorcluster)
        n208 = shared-variable "RT CompactRIO Target\\RT_EPICS_Shared_Variables.lvlib\\2iddVELO:VP:Scanning"(w584) -> ()  [unwired: 1 in, 1 out]
      }
      frame "Fly Scanning" {
        w635 = "%8f"  # format string
        w634 = ","  # delimiter (Tab)
        w662 = 0.0  # t0
        # "This creates time gap between subsequent\n reads in order to fill FIFO"
        n209 = xnode "Read/Write Control"("FPGA VI Reference In"=w640, "error in"=w654) -> ("FPGA VI Reference Out"=w625:refnum<k20>, "error out"=w624:errorcluster, "Number of Data Strings"=→"Number of Data Strings":i32, "FPGA state"=w619:T10)
        n210 = local read "Datalog Time Period (uSec)"() -> (w660:u32)
        n211 = Not Equal?(x=T10."Run", y=w619) -> (x != y?=w616:bool)
        n212 = Multiply(x=1e-06, y=w660) -> (x*y=w657:dbl)
        "Datalog Time Period (sec)" <- w657
        n213 = local read "Trigger Frequency (Hz)"() -> (w597:dbl)
        n214 = xnode "Invoke Method"("FPGA VI Reference In"=w625, "error in"=w624, "Number of Elements"=u32 0, "Timeout (ms)"=0) -> ("FPGA VI Reference Out"=w622:refnum<k20>, "error out"=w623:errorcluster, "Elements Remaining"=w601:u32)  [unwired: 1 out]
        n215 = Divide(x=1.0, y=w657) -> (x/y=w628:dbl)
        "Datalog Rate (Hz)" <- w628
        n216 = Multiply(x="FIFO Time Period", y=w628) -> (x*y=w598:dbl)
        n217 = Multiply(x=w598, y=5 ("Number of Data Strings 2")) -> (x*y=w626:dbl)
        n218 = To Unsigned Long Integer(number=w626) -> (unsigned 32bit integer=w621:u32)
        "Number of Elements" <- w621
        n219 = Divide(x=w597, y=w598) -> (x/y=w596:dbl)
        n220 = Divide(x=i16 1000, y=w596) -> (x/y=w594:dbl)
        n221 = Max & Min(x=w601, y=w621) -> (min(x,y)=w600:u32)  [unwired: 1 out]
        "Elements Available in FIFO" <- w600
        n222 = Equal?(x=u32 0, y=w601) -> (x = y?=w617:bool)
        n223 = And(x=w616, y=w617) -> (x .and. y?=w615:bool)
        n224 = xnode "Invoke Method"("FPGA VI Reference In"=w622, "error in"=w623, "Number of Elements"=w600, "Timeout (ms)"="Timeout (ms)") -> ("FPGA VI Reference Out"=w639:refnum<k20>, "error out"=w638:errorcluster, "Data"=w656:fxp<+/-,58,25>[], "Elements Remaining"=→"Elements Remaining" →"Elements Remaining in FIFO":u32)
        "Data" <- w656
        n225 = Decimate 1D Array(w656) -> (w611:fxp<+/-,58,25>[], w610:fxp<+/-,58,25>[], w609:fxp<+/-,58,25>[], w608:fxp<+/-,58,25>[], w641:fxp<+/-,58,25>[])
        n226 = To Quad Integer(1:w594) -> (0:w593:i64)
        n227 = Build Array(w611, w610, w609, w608, w641) -> (w663:fxp<+/-,58,25>[][])
        n228 = To Double Precision Float(number=w663) -> (double precision float=w658:dbl[][])
        n229 = Transpose 2D Array(2D array=w658) -> (transposed array=w653:dbl[][])